vi "SaccadeAnalyser - Main.vi"(8 "error in (no error)":errorcluster, 11 "Data IN":T3={"Impulse Positions"=[{"Start"=5471, "End"=5813, "Impulse Plane"=enum."Yaw", "Impulse Direction +ve?"=FALSE, "Time offset"=0, "Amplitude offset"=0.0}, {"Start"=6974, "End"=7325, "Impulse Plane"=enum."Yaw", "Impulse Direction +ve?"=TRUE, "Time offset"=0, "Amplitude offset"=0.0}, {"Start"=7641, "End"=7980, "Impulse Plane"=enum."Yaw", "Impulse Direction +ve?"=FALSE, "Time offset"=0, "Amplitude offset"=0.0}, {"Start"=9060, "End"=9400, "Impulse Plane"=enum."Yaw", "Impulse Direction +ve?"=FALSE, "Time offset"=0, "Amplitude offset"=0.0}, {"Start"=9938, "End"=10282, "Impulse Plane"=enum."Yaw", "Impulse Direction +ve?"=FALSE, "Time offset"=0, "Amplitude offset"=0.0}, {"Start"=10800, "End"=11142, "Impulse Plane"=enum."Yaw", "Impulse Direction +ve?"=FALSE, "Time offset"=0, "Amplitude offset"=0.0}, {"Start"=11602, "End"=11942, "Impulse Plane"=enum."Yaw", "Impulse Direction +ve?"=TRUE, "Time offset"=0, "Amplitude offset"=0.0}, {"Start"=12449, "End"=12790, "Impulse Plane"=enum."Yaw", "Impulse Direction +ve?"=TRUE, "Time offset"=0, "Amplitude offset"=0.0}, {"Start"=13310, "End"=13653, "Impulse Plane"=enum."Yaw", "Impulse Direction +ve?"=TRUE, "Time offset"=0, "Amplitude offset"=0.0}, {"Start"=14191, "End"=14535, "Impulse Plane"=enum."Yaw", "Impulse Direction +ve?"=TRUE, "Time offset"=0, "Amplitude offset"=0.0}, {"Start"=15040, "End"=15380, "Impulse Plane"=enum."Yaw", "Impulse Direction +ve?"=FALSE, "Time offset"=0, "Amplitude offset"=0.0}, {"Start"=16780, "End"=17124, "Impulse Plane"=enum."Yaw", "Impulse Direction +ve?"=TRUE, "Time offset"=0, "Amplitude offset"=0.0}, {"Start"=17572, "End"=17913, "Impulse Plane"=enum."Yaw", "Impulse Direction +ve?"=FALSE, "Time offset"=0, "Amplitude offset"=0.0}, {"Start"=18369, "End"=18713, "Impulse Plane"=enum."Yaw", "Impulse Direction +ve?"=FALSE, "Time offset"=0, "Amplitude offset"=0.0}, {"Start"=19174, "End"=19519, "Impulse Plane"=enum."Yaw", "Impulse Direction +ve?"=FALSE, "Time offset"=0, "Amplitude offset"=0.0}, {"Start"=19928, "End"=20270, "Impulse Plane"=enum."Yaw", "Impulse Direction +ve?"=TRUE, "Time offset"=0, "Amplitude offset"=0.0}, {"Start"=20762, "End"=21121, "Impulse Plane"=enum."Yaw", "Impulse Direction +ve?"=FALSE, "Time offset"=0, "Amplitude offset"=0.0}, {"Start"=21554, "End"=21888, "Impulse Plane"=enum."Yaw", "Impulse Direction +ve?"=FALSE, "Time offset"=0, "Amplitude offset"=0.0}, {"Start"=22293, "End"=22639, "Impulse Plane"=enum."Yaw", "Impulse Direction +ve?"=TRUE, "Time offset"=0, "Amplitude offset"=0.0}, {"Start"=23109, "End"=23464, "Impulse Plane"=enum."Yaw", "Impulse Direction +ve?"=TRUE, "Time offset"=0, "Amplitude offset"=0.0}, {"Start"=23868, "End"=24215, "Impulse Plane"=enum."Yaw", "Impulse Direction +ve?"=TRUE, "Time offset"=0, "Amplitude offset"=0.0}, {"Start"=24643, "End"=24992, "Impulse Plane"=enum."Yaw", "Impulse Direction +ve?"=FALSE, "Time offset"=0, "Amplitude offset"=0.0}, {"Start"=25685, "End"=26023, "Impulse Plane"=enum."Yaw", "Impulse Direction +ve?"=FALSE, "Time offset"=0, "Amplitude offset"=0.0}, {"Start"=26431, "End"=26768, "Impulse Plane"=enum."Yaw", "Impulse Direction +ve?"=FALSE, "Time offset"=0, "Amplitude offset"=0.0}, {"Start"=27251, "End"=27595, "Impulse Plane"=enum."Yaw", "Impulse Direction +ve?"=FALSE, "Time offset"=0, "Amplitude offset"=0.0}, {"Start"=28832, "End"=29180, "Impulse Plane"=enum."Yaw", "Impulse Direction +ve?"=TRUE, "Time offset"=0, "Amplitude offset"=0.0}, {"Start"=31028, "End"=31383, "Impulse Plane"=enum."LARP", "Impulse Direction +ve?"=FALSE, "Time offset"=0, "Amplitude offset"=0.0}, {"Start"=32603, "End"=32936, "Impulse Plane"=enum."LARP", "Impulse Direction +ve?"=TRUE, "Time offset"=0, "Amplitude offset"=0.0}, {"Start"=33445, "End"=33779, "Impulse Plane"=enum."LARP", "Impulse Direction +ve?"=TRUE, "Time offset"=0, "Amplitude offset"=0.0}, {"Start"=34276, "End"=34629, "Impulse Plane"=enum."LARP", "Impulse Direction +ve?"=FALSE, "Time offset"=0, "Amplitude offset"=0.0}, {"Start"=35114, "End"=35460, "Impulse Plane"=enum."LARP", "Impulse Direction +ve?"=FALSE, "Time offset"=0, "Amplitude offset"=0.0}, {"Start"=35981, "End"=36324, "Impulse Plane"=enum."LARP", "Impulse Direction +ve?"=TRUE, "Time offset"=0, "Amplitude offset"=0.0}, {"Start"=36920, "End"=37249, "Impulse Plane"=enum."LARP", "Impulse Direction +ve?"=TRUE, "Time offset"=0, "Amplitude offset"=0.0}, {"Start"=37988, "End"=38322, "Impulse Plane"=enum."LARP", "Impulse Direction +ve?"=TRUE, "Time offset"=0, "Amplitude offset"=0.0}, {"Start"=38964, "End"=39324, "Impulse Plane"=enum."LARP", "Impulse Direction +ve?"=FALSE, "Time offset"=0, "Amplitude offset"=0.0}, {"Start"=39948, "End"=40284, "Impulse Plane"=enum."LARP", "Impulse Direction +ve?"=TRUE, "Time offset"=0, "Amplitude offset"=0.0}, {"Start"=40958, "End"=41293, "Impulse Plane"=enum."LARP", "Impulse Direction +ve?"=TRUE, "Time offset"=0, "Amplitude offset"=0.0}, {"Start"=41899, "End"=42229, "Impulse Plane"=enum."LARP", "Impulse Direction +ve?"=TRUE, "Time offset"=0, "Amplitude offset"=0.0}, {"Start"=42801, "End"=43154, "Impulse Plane"=enum."LARP", "Impulse Direction +ve?"=FALSE, "Time offset"=0, "Amplitude offset"=0.0}, {"Start"=43641, "End"=43980, "Impulse Plane"=enum."LARP", "Impulse Direction +ve?"=TRUE, "Time offset"=0, "Amplitude offset"=0.0}, {"Start"=44466, "End"=44821, "Impulse Plane"=enum."LARP", "Impulse Direction +ve?"=FALSE, "Time offset"=0, "Amplitude offset"=0.0}, {"Start"=45388, "End"=45722, "Impulse Plane"=enum."LARP", "Impulse Direction +ve?"=TRUE, "Time offset"=0, "Amplitude offset"=0.0}, {"Start"=46149, "End"=46510, "Impulse Plane"=enum."LARP", "Impulse Direction +ve?"=FALSE, "Time offset"=0, "Amplitude offset"=0.0}, {"Start"=47874, "End"=48206, "Impulse Plane"=enum."LARP", "Impulse Direction +ve?"=TRUE, "Time offset"=0, "Amplitude offset"=0.0}, {"Start"=50143, "End"=50479, "Impulse Plane"=enum."RALP", "Impulse Direction +ve?"=TRUE, "Time offset"=0, "Amplitude offset"=0.0}, {"Start"=50976, "End"=51310, "Impulse Plane"=enum."RALP", "Impulse Direction +ve?"=FALSE, "Time offset"=0, "Amplitude offset"=0.0}, {"Start"=51892, "End"=52226, "Impulse Plane"=enum."RALP", "Impulse Direction +ve?"=FALSE, "Time offset"=0, "Amplitude offset"=0.0}, {"Start"=52839, "End"=53171, "Impulse Plane"=enum."RALP", "Impulse Direction +ve?"=FALSE, "Time offset"=0, "Amplitude offset"=0.0}, {"Start"=53676, "End"=54012, "Impulse Plane"=enum."RALP", "Impulse Direction +ve?"=TRUE, "Time offset"=0, "Amplitude offset"=0.0}, {"Start"=54530, "End"=54877, "Impulse Plane"=enum."RALP", "Impulse Direction +ve?"=FALSE, "Time offset"=0, "Amplitude offset"=0.0}, {"Start"=55371, "End"=55711, "Impulse Plane"=enum."RALP", "Impulse Direction +ve?"=TRUE, "Time offset"=0, "Amplitude offset"=0.0}, {"Start"=56153, "End"=56482, "Impulse Plane"=enum."RALP", "Impulse Direction +ve?"=FALSE, "Time offset"=0, "Amplitude offset"=0.0}, {"Start"=57053, "End"=57390, "Impulse Plane"=enum."RALP", "Impulse Direction +ve?"=FALSE, "Time offset"=0, "Amplitude offset"=0.0}, {"Start"=57954, "End"=58292, "Impulse Plane"=enum."RALP", "Impulse Direction +ve?"=FALSE, "Time offset"=0, "Amplitude offset"=0.0}, {"Start"=58794, "End"=59130, "Impulse Plane"=enum."RALP", "Impulse Direction +ve?"=TRUE, "Time offset"=0, "Amplitude offset"=0.0}, {"Start"=59587, "End"=59931, "Impulse Plane"=enum."RALP", "Impulse Direction +ve?"=TRUE, "Time offset"=0, "Amplitude offset"=0.0}, {"Start"=60399, "End"=60744, "Impulse Plane"=enum."RALP", "Impulse Direction +ve?"=FALSE, "Time offset"=0, "Amplitude offset"=0.0}, {"Start"=61218, "End"=61559, "Impulse Plane"=enum."RALP", "Impulse Direction +ve?"=FALSE, "Time offset"=0, "Amplitude offset"=0.0}, {"Start"=62100, "End"=62442, "Impulse Plane"=enum."RALP", "Impulse Direction +ve?"=FALSE, "Time offset"=0, "Amplitude offset"=0.0}, {"Start"=62989, "End"=63322, "Impulse Plane"=enum."RALP", "Impulse Direction +ve?"=FALSE, "Time offset"=0, "Amplitude offset"=0.0}, {"Start"=63787, "End"=64136, "Impulse Plane"=enum."RALP", "Impulse Direction +ve?"=TRUE, "Time offset"=0, "Amplitude offset"=0.0}, {"Start"=64603, "End"=64953, "Impulse Plane"=enum."RALP", "Impulse Direction +ve?"=FALSE, "Time offset"=0, "Amplitude offset"=0.0}, {"Start"=65462, "End"=65795, "Impulse Plane"=enum."RALP", "Impulse Direction +ve?"=FALSE, "Time offset"=0, "Amplitude offset"=0.0}, {"Start"=66308, "End"=66645, "Impulse Plane"=enum."RALP", "Impulse Direction +ve?"=FALSE, "Time offset"=0, "Amplitude offset"=0.0}, {"Start"=67052, "End"=67402, "Impulse Plane"=enum."RALP", "Impulse Direction +ve?"=TRUE, "Time offset"=0, "Amplitude offset"=0.0}], "No. Imp"=15, "Parameter Time Series"=[{"time offset"=0.0, "Offset"=0.0, "Gain"=1.0, "inverse"=FALSE, "filter data"=FALSE, "dots"=FALSE, "interpolate"=FALSE, "List 1"=5, "Color Box"=6618880, "Boolean"=TRUE}, {"time offset"=0.0, "Offset"=0.0, "Gain"=1.0, "inverse"=FALSE, "filter data"=FALSE, "dots"=FALSE, "interpolate"=FALSE, "List 1"=6, "Color Box"=6618880, "Boolean"=FALSE}, {"time offset"=0.0, "Offset"=0.0, "Gain"=1.0, "inverse"=FALSE, "filter data"=FALSE, "dots"=FALSE, "interpolate"=FALSE, "List 1"=7, "Color Box"=6618880, "Boolean"=FALSE}, {"time offset"=0.0, "Offset"=0.0, "Gain"=1.0, "inverse"=FALSE, "filter data"=FALSE, "dots"=FALSE, "interpolate"=FALSE, "List 1"=13, "Color Box"=16777224, "Boolean"=TRUE}, {"time offset"=0.0, "Offset"=0.0, "Gain"=1.0, "inverse"=FALSE, "filter data"=FALSE, "dots"=FALSE, "interpolate"=FALSE, "List 1"=14, "Color Box"=16777224, "Boolean"=FALSE}, {"time offset"=0.0, "Offset"=0.0, "Gain"=1.0, "inverse"=FALSE, "filter data"=FALSE, "dots"=FALSE, "interpolate"=FALSE, "List 1"=15, "Color Box"=16777224, "Boolean"=FALSE}], "Parameter Impuls Series"=[{"Color"=6618880, "Visible"=TRUE, "Channel"=1, "Invert"=FALSE, "Desaccade"=FALSE, "Offset"=0.0, "Gain"=1.0}, {"Color"=6618880, "Visible"=FALSE, "Channel"=6, "Invert"=FALSE, "Desaccade"=FALSE, "Offset"=0.0, "Gain"=1.0}, {"Color"=6618880, "Visible"=FALSE, "Channel"=7, "Invert"=FALSE, "Desaccade"=FALSE, "Offset"=0.0, "Gain"=1.0}, {"Color"=16777224, "Visible"=TRUE, "Channel"=13, "Invert"=FALSE, "Desaccade"=FALSE, "Offset"=0.0, "Gain"=1.0}, {"Color"=16777224, "Visible"=FALSE, "Channel"=14, "Invert"=FALSE, "Desaccade"=FALSE, "Offset"=0.0, "Gain"=1.0}, {"Color"=16777224, "Visible"=FALSE, "Channel"=15, "Invert"=FALSE, "Desaccade"=FALSE, "Offset"=0.0, "Gain"=1.0}], "Experiment Parameters"={"Freq"=0.0, "Vel"=0, "Acc"=0, "Stimulus"="Head Impulse"}, "Autosort File"=refnum, "Data File"={"Data Channels"=array34x71049[2415666 elements], "Sample Rate"=500, "Channel List"=["Hz Position-in-Head", "Hz Velocity-in-Head", "Hy Position-in-Head", "Hy Velocity-in-Head", "Hx Position-in-Head", "Hx Velocity-in-Head", "Hl Velocity-in-Head", "Hr Velocity-in-Head", "Lx Position-in-Head", "Ly Position-in-Head", "Lz Position-in-Head", "Lx Velocity-in-Head", "Ly Velocity-in-Head", "Lz Velocity-in-Head", "Ll Velocity-in-Head", "Lr Velocity-in-Head", "Rx Position-in-Head", "Ry Position-in-Head", "Rz Position-in-Head", "Rx Velocity-in-Head", "Ry Velocity-in-Head", "Rz Velocity-in-Head", "Rl Velocity-in-Head", "Rr Velocity-in-Head", "Target on/off", "aux input 1", "aux input 2", " ", "", "", "", "Target Hor", "Target Ver", ""]}, "Experiment data path"=path "C:/Users/w.figtree/Desktop/Coils Data/3", "Image data path"=path "/Macintosh HD/Users/patrick/Studium/Diploma Thesis/Data Analysis", "LVS data path"=path "/Macintosh HD/Users/patrick/Studium/Diploma Thesis/Data Analysis", "Raw copy path"=path "/Macintosh HD/Users/patrick/Studium/Diploma Thesis/Data Analysis", "filename"="passive_lvs.lvs", "desaccading parameters"={"Tolerance"=3, "Acc Range"=7000.0, "Sample Rate"=500, "Impulse Plane 2"=enum."Yaw", "Impulse dir"=FALSE}, "Experiment Parameters 2"={"Subject"="SE Trial Short Term", "Strain"="", "Rotation plane"="", "Experimenter"=" ", "Trial"=0.0, "Time"=0.0}, "Excel"={"Excel._Application"=refnum, "Use Excel"=TRUE, "Worksheet SINE"=refnum, "Row SINE"=0, "Worksheet TRANS"=refnum, "Row TRANS"=0}, "Session Config File"=refnum, "Autosort Parameter Set"=4, "EMA Version"="EMA 2016a", "desacc "={"Threshold 1 [Acc]"=7000.0, "Threshold 2 [% of TH1]"=60, "tolerance"=3, "Search WD "=0.1, " always use TH2"=FALSE, "Range"=3.0, "Max time"=120.0, "Min time"=20.0, "Velocity Threshold"=150}, "Cycle Nr for Saccades"={"POS"=0, "NEG"=0}, "calibration name"="u_calibration_1_p00001s001_calib.mat", "Excel"=refnum} {"Parameter Time Series"."time offset" format="%.3f"; "Parameter Time Series"."Gain" format="%.1f"; "Parameter Time Series"."Offset" format="%.1f"; "Parameter Time Series"."List 1" items=["Motor-Pos", "Motor-Vel", "Lx Position-in-Head", "Ly Position-in-Head", "Lz Position-in-Head", "Lx Velocity-in-Head", "Ly Velocity-in-Head", "Lz Velocity-in-Head", "Ll Velocity-in-Head", "Lr Velocity-in-Head", "Lx Accel-in-Head", "Ly Accel-in-Head", "Lz Accel-in-Head", "Rx Position-in-Head", "Ry Position-in-Head", "Rz Position-in-Head", "Rx Velocity-in-Head", "Ry Velocity-in-Head", "Rz Velocity-in-Head", "Rl Velocity-in-Head", "Rr Velocity-in-Head", "Rx Accel-in-Head", "Ry Accel-in-Head", "Rz Accel-in-Head", "Global Trigger", "", "", ""]; "Parameter Impuls Series"."Gain" format="%.1f"; "Parameter Impuls Series"."Offset" format="%.1f"}) -> (0 "error out":errorcluster, 3 "Data OUT":T3={"Impulse Positions"=[{"Start"=5471, "End"=5813, "Impulse Plane"=enum."Yaw", "Impulse Direction +ve?"=FALSE, "Time offset"=0, "Amplitude offset"=0.0}, {"Start"=6974, "End"=7325, "Impulse Plane"=enum."Yaw", "Impulse Direction +ve?"=TRUE, "Time offset"=0, "Amplitude offset"=0.0}, {"Start"=7641, "End"=7980, "Impulse Plane"=enum."Yaw", "Impulse Direction +ve?"=FALSE, "Time offset"=0, "Amplitude offset"=0.0}, {"Start"=9060, "End"=9400, "Impulse Plane"=enum."Yaw", "Impulse Direction +ve?"=FALSE, "Time offset"=0, "Amplitude offset"=0.0}, {"Start"=9938, "End"=10282, "Impulse Plane"=enum."Yaw", "Impulse Direction +ve?"=FALSE, "Time offset"=0, "Amplitude offset"=0.0}, {"Start"=10800, "End"=11142, "Impulse Plane"=enum."Yaw", "Impulse Direction +ve?"=FALSE, "Time offset"=0, "Amplitude offset"=0.0}, {"Start"=11602, "End"=11942, "Impulse Plane"=enum."Yaw", "Impulse Direction +ve?"=TRUE, "Time offset"=0, "Amplitude offset"=0.0}, {"Start"=12449, "End"=12790, "Impulse Plane"=enum."Yaw", "Impulse Direction +ve?"=TRUE, "Time offset"=0, "Amplitude offset"=0.0}, {"Start"=13310, "End"=13653, "Impulse Plane"=enum."Yaw", "Impulse Direction +ve?"=TRUE, "Time offset"=0, "Amplitude offset"=0.0}, {"Start"=14191, "End"=14535, "Impulse Plane"=enum."Yaw", "Impulse Direction +ve?"=TRUE, "Time offset"=0, "Amplitude offset"=0.0}, {"Start"=15040, "End"=15380, "Impulse Plane"=enum."Yaw", "Impulse Direction +ve?"=FALSE, "Time offset"=0, "Amplitude offset"=0.0}, {"Start"=16780, "End"=17124, "Impulse Plane"=enum."Yaw", "Impulse Direction +ve?"=TRUE, "Time offset"=0, "Amplitude offset"=0.0}, {"Start"=17572, "End"=17913, "Impulse Plane"=enum."Yaw", "Impulse Direction +ve?"=FALSE, "Time offset"=0, "Amplitude offset"=0.0}, {"Start"=18369, "End"=18713, "Impulse Plane"=enum."Yaw", "Impulse Direction +ve?"=FALSE, "Time offset"=0, "Amplitude offset"=0.0}, {"Start"=19174, "End"=19519, "Impulse Plane"=enum."Yaw", "Impulse Direction +ve?"=FALSE, "Time offset"=0, "Amplitude offset"=0.0}, {"Start"=19928, "End"=20270, "Impulse Plane"=enum."Yaw", "Impulse Direction +ve?"=TRUE, "Time offset"=0, "Amplitude offset"=0.0}, {"Start"=20762, "End"=21121, "Impulse Plane"=enum."Yaw", "Impulse Direction +ve?"=FALSE, "Time offset"=0, "Amplitude offset"=0.0}, {"Start"=21554, "End"=21888, "Impulse Plane"=enum."Yaw", "Impulse Direction +ve?"=FALSE, "Time offset"=0, "Amplitude offset"=0.0}, {"Start"=22293, "End"=22639, "Impulse Plane"=enum."Yaw", "Impulse Direction +ve?"=TRUE, "Time offset"=0, "Amplitude offset"=0.0}, {"Start"=23109, "End"=23464, "Impulse Plane"=enum."Yaw", "Impulse Direction +ve?"=TRUE, "Time offset"=0, "Amplitude offset"=0.0}, {"Start"=23868, "End"=24215, "Impulse Plane"=enum."Yaw", "Impulse Direction +ve?"=TRUE, "Time offset"=0, "Amplitude offset"=0.0}, {"Start"=24643, "End"=24992, "Impulse Plane"=enum."Yaw", "Impulse Direction +ve?"=FALSE, "Time offset"=0, "Amplitude offset"=0.0}, {"Start"=25685, "End"=26023, "Impulse Plane"=enum."Yaw", "Impulse Direction +ve?"=FALSE, "Time offset"=0, "Amplitude offset"=0.0}, {"Start"=26431, "End"=26768, "Impulse Plane"=enum."Yaw", "Impulse Direction +ve?"=FALSE, "Time offset"=0, "Amplitude offset"=0.0}, {"Start"=27251, "End"=27595, "Impulse Plane"=enum."Yaw", "Impulse Direction +ve?"=FALSE, "Time offset"=0, "Amplitude offset"=0.0}, {"Start"=28832, "End"=29180, "Impulse Plane"=enum."Yaw", "Impulse Direction +ve?"=TRUE, "Time offset"=0, "Amplitude offset"=0.0}, {"Start"=31028, "End"=31383, "Impulse Plane"=enum."LARP", "Impulse Direction +ve?"=FALSE, "Time offset"=0, "Amplitude offset"=0.0}, {"Start"=32603, "End"=32936, "Impulse Plane"=enum."LARP", "Impulse Direction +ve?"=TRUE, "Time offset"=0, "Amplitude offset"=0.0}, {"Start"=33445, "End"=33779, "Impulse Plane"=enum."LARP", "Impulse Direction +ve?"=TRUE, "Time offset"=0, "Amplitude offset"=0.0}, {"Start"=34276, "End"=34629, "Impulse Plane"=enum."LARP", "Impulse Direction +ve?"=FALSE, "Time offset"=0, "Amplitude offset"=0.0}, {"Start"=35114, "End"=35460, "Impulse Plane"=enum."LARP", "Impulse Direction +ve?"=FALSE, "Time offset"=0, "Amplitude offset"=0.0}, {"Start"=35981, "End"=36324, "Impulse Plane"=enum."LARP", "Impulse Direction +ve?"=TRUE, "Time offset"=0, "Amplitude offset"=0.0}, {"Start"=36920, "End"=37249, "Impulse Plane"=enum."LARP", "Impulse Direction +ve?"=TRUE, "Time offset"=0, "Amplitude offset"=0.0}, {"Start"=37988, "End"=38322, "Impulse Plane"=enum."LARP", "Impulse Direction +ve?"=TRUE, "Time offset"=0, "Amplitude offset"=0.0}, {"Start"=38964, "End"=39324, "Impulse Plane"=enum."LARP", "Impulse Direction +ve?"=FALSE, "Time offset"=0, "Amplitude offset"=0.0}, {"Start"=39948, "End"=40284, "Impulse Plane"=enum."LARP", "Impulse Direction +ve?"=TRUE, "Time offset"=0, "Amplitude offset"=0.0}, {"Start"=40958, "End"=41293, "Impulse Plane"=enum."LARP", "Impulse Direction +ve?"=TRUE, "Time offset"=0, "Amplitude offset"=0.0}, {"Start"=41899, "End"=42229, "Impulse Plane"=enum."LARP", "Impulse Direction +ve?"=TRUE, "Time offset"=0, "Amplitude offset"=0.0}, {"Start"=42801, "End"=43154, "Impulse Plane"=enum."LARP", "Impulse Direction +ve?"=FALSE, "Time offset"=0, "Amplitude offset"=0.0}, {"Start"=43641, "End"=43980, "Impulse Plane"=enum."LARP", "Impulse Direction +ve?"=TRUE, "Time offset"=0, "Amplitude offset"=0.0}, {"Start"=44466, "End"=44821, "Impulse Plane"=enum."LARP", "Impulse Direction +ve?"=FALSE, "Time offset"=0, "Amplitude offset"=0.0}, {"Start"=45388, "End"=45722, "Impulse Plane"=enum."LARP", "Impulse Direction +ve?"=TRUE, "Time offset"=0, "Amplitude offset"=0.0}, {"Start"=46149, "End"=46510, "Impulse Plane"=enum."LARP", "Impulse Direction +ve?"=FALSE, "Time offset"=0, "Amplitude offset"=0.0}, {"Start"=47874, "End"=48206, "Impulse Plane"=enum."LARP", "Impulse Direction +ve?"=TRUE, "Time offset"=0, "Amplitude offset"=0.0}, {"Start"=50143, "End"=50479, "Impulse Plane"=enum."RALP", "Impulse Direction +ve?"=TRUE, "Time offset"=0, "Amplitude offset"=0.0}, {"Start"=50976, "End"=51310, "Impulse Plane"=enum."RALP", "Impulse Direction +ve?"=FALSE, "Time offset"=0, "Amplitude offset"=0.0}, {"Start"=51892, "End"=52226, "Impulse Plane"=enum."RALP", "Impulse Direction +ve?"=FALSE, "Time offset"=0, "Amplitude offset"=0.0}, {"Start"=52839, "End"=53171, "Impulse Plane"=enum."RALP", "Impulse Direction +ve?"=FALSE, "Time offset"=0, "Amplitude offset"=0.0}, {"Start"=53676, "End"=54012, "Impulse Plane"=enum."RALP", "Impulse Direction +ve?"=TRUE, "Time offset"=0, "Amplitude offset"=0.0}, {"Start"=54530, "End"=54877, "Impulse Plane"=enum."RALP", "Impulse Direction +ve?"=FALSE, "Time offset"=0, "Amplitude offset"=0.0}, {"Start"=55371, "End"=55711, "Impulse Plane"=enum."RALP", "Impulse Direction +ve?"=TRUE, "Time offset"=0, "Amplitude offset"=0.0}, {"Start" (continued)
-54.18247144797069, -58.85281689160722, -63.91527138905126, -69.3816768064082, -75.22429125556431, -81.37762698666069, -87.75180274500077, -94.23796057331468, -100.71571205715665, -107.07112629665112, -113.2080026001733, -119.04423669102385, -124.52204306435647, -129.6179037571645, -134.3434864691834, -138.73926124919257, -142.86209314608806, -146.77852632236662, -150.55410864602925, -154.2421058778206, -157.8608435457303, -161.38556543542902, -164.75519586867193, -167.878112041269, -170.6502845196639, -172.96947690993014, -174.74780026444301, -175.9280234619177, -176.49581974428241, -176.47783870432215, -175.92566673674776, -174.9055756754708, -173.49760575715453, -171.7834624665382, -169.83161630071703, -167.69551193456192, -165.41647407002708, -163.02092536825774, -160.50399517975018, -157.8263795045505, -154.92869248428667, -151.7392178656919, -148.18363503277277, -144.19520813467358, -139.7423154139475, -134.85092284147765, -129.5970332835845, -124.096932573479, -118.48663287415354, -112.89326377420801, -107.41192289509742, -102.09133956405964, -96.91932930045344, -91.82924084415812, -86.72929490339284, -81.52158361787951, -76.1282941909947, -70.50762789188907, -64.66023923119536, -58.64052733673002, -52.54018902245833, -46.45809012434801, -40.486829092171924, -34.70668063780862, -29.173216331551032, -23.9068786063661, -18.897099148136192, -14.114118816191809, -9.520293557801804, -5.085847473387664, -0.7981606818145077, 3.3266043290818934, 7.243600002532165, 10.885420249895338, 14.161767360680157, 16.984238540492136, 19.291750959591102, 21.063902044408295, 22.331979940494904, 23.17761342325074, 23.721961474588795, 24.112784288313726, 24.491300668844953, 24.954722286655777, 25.548108319995535, 26.25835502219787, 27.009352039914436, 27.685557314658922, 28.168888441777447, 28.373084425112715, 28.259535186152696, 27.842133775360793, 27.188150755230232, 26.406250500356492, 25.615461263548987, 24.910485897492496, 24.346023233855814, 23.92691315712331, 23.608231595379664, 23.316584778717154, 22.97439243815799, 22.516811117961932, 21.918073580662337, 21.199324383617018, 20.41268969980475, 19.630359806325515, 18.925688883278173, 18.35445806189755, 17.94200024522094, 17.668844949225154, 17.48230912370444, 17.320743177459768, 17.12385592094169, 16.848651342354945, 16.48521549632595, 16.053715760638944, 15.599731481783138, 15.187115328471895, 14.872560249314708, 14.690476111081628, 14.654617574216875, 14.750456991166905, 14.93679615927241, 15.155141464873388, 15.333160190841902, 15.398738035467435, 15.29496106484143, 14.988709233052518, 14.477914274794113, 13.791715142798871, 12.98608736614728, 12.143907008543643, 11.359534797804809, 10.712039410503696, 10.254402747409266, 9.996473345954591, 9.896879988642478, 9.883403069720273, 9.859589516965436, 9.721973952789982, 9.396474330493742, 8.8572878573063, 8.126364534227164, 7.264175814803053, 6.355998470318044, 5.489439194352843, 4.7331879614108505, 4.122707511796716, 3.65264371887878, 3.286290193278276, 2.9766469769695836, 2.680197842403923, 2.3715537962781688, 2.054470430273149, 1.7588126482498483, 1.52762158204097, 1.3969988798953015, 1.3837046107842852, 1.4780084889263279, 1.6331366871599418, 1.7862480312450515, 1.885768730098075, 1.8964541688469012, 1.8162169165165416, 1.6814817264069895, 1.5492834774423194, 1.484862531012908, 1.5421064788750378, 1.7350747823148893, 2.0342448608033195, 2.379446691066832, 2.6948282712623737, 2.911116060608993, 2.9842378047308706, 2.9083083080686016, 2.7160208417143217, 2.4711098156462157, 2.256715447981385, 2.148013016215092, 2.187585248222959, 2.3803037826910867, 2.6983328403827826, 3.0862430081882692, 3.4771760047328684, 3.8144998017781937, 4.063608708587875, 4.220732678012546, 4.314758958249271, 4.385161364394381, 4.451563149829603, 4.516553485433068, 4.5711222556517725, 4.5789244340039374, 4.495990520342794, 4.300879185323019, 3.999300290032796, 3.6267710749586684, 3.2456696612949933, 2.9267834631551075, 2.7279329460099753, 2.6791526464304543, 2.764403437378572, 2.924982772356076, 3.0845635011921093, 3.1660247683184704, 3.1140733546638995, 2.9142235252131066, 2.6045926121551446, 2.264439578758724, 1.9827108041327461, 1.8446572231616623, 1.9016973069974075, 2.1477989186114366, 2.527543767369518, 2.9494945166396676, 3.316294504066529, 3.554920234020117, 3.6294412691334976, 3.5518308896879076, 3.381651807861633, 3.1987672126172613, 3.0794265856609844, 3.076618052634122, 3.2028855967548573, 3.4357915499468694, 3.7262128069143348, 4.011008721689602, 4.241013746798439, 4.4004494908201375, 4.501263210760912, 4.57564361728543, 4.674574896548988, 4.847554015003683, 5.118620024272339, 5.476792247776838, 5.882038540567098, 6.280337746221127, 6.610772610856507, 6.824568969574903, 6.902440280843165, 6.859370359784798, 6.743336212454451, 6.611463939269871, 6.5152928701361645]}, {[0.0, 2.0, 4.0, 6.0, 8.0, 10.0, 12.0, 14.0, 16.0, 18.000000000000004, 20.0, 22.0, 24.0, 26.000000000000004, 28.0, 30.0, 32.0, 34.0, 36.00000000000001, 38.0, 40.0, 42.0, 44.0, 46.0, 48.0, 50.0, 52.00000000000001, 54.0, 56.0, 58.0, 60.0, 62.0, 64.0, 66.0, 68.0, 70.0, 72.00000000000001, 74.0, 76.0, 78.0, 80.0, 82.0, 84.0, 86.0, 88.0, 90.0, 92.0, 94.0, 96.0, 98.0, 100.0, 102.00000000000001, 104.00000000000001, 106.0, 108.0, 110.0, 112.0, 114.0, 116.0, 118.00000000000001, 120.0, 122.0, 124.0, 126.0, 128.0, 130.0, 132.0, 134.0, 136.0, 138.0, 140.0, 142.00000000000003, 144.00000000000003, 146.0, 148.0, 150.0, 152.0, 154.0, 156.0, 158.0, 160.0, 162.0, 164.0, 166.0, 168.0, 170.0, 172.0, 174.00000000000003, 176.0, 178.0, 180.0, 182.0, 184.0, 186.0, 188.0, 190.0, 192.0, 194.0, 196.0, 198.0, 200.0, 202.0, 204.00000000000003, 206.00000000000003, 208.00000000000003, 210.0, 212.0, 214.0, 216.0, 218.0, 220.0, 222.0, 224.0, 226.0, 228.0, 230.0, 232.0, 234.0, 236.00000000000003, 238.00000000000003, 240.0, 242.0, 244.0, 246.0, 248.0, 250.0, 252.0, 254.0, 256.0, 258.0, 260.0, 262.0, 264.0, 266.0, 268.0, 270.0, 272.0, 274.0, 276.0, 278.0, 280.0, 282.0, 284.00000000000006, 286.00000000000006, 288.00000000000006, 290.0, 292.0, 294.0, 296.0, 298.0, 300.0, 302.0, 304.0, 306.0, 308.0, 310.0, 312.0, 314.0, 316.0, 318.0, 320.0, 322.0, 324.0, 326.0, 328.0, 330.0, 332.0, 334.0, 336.0, 338.0, 340.0, 342.0, 344.0, 346.00000000000006, 348.00000000000006, 350.00000000000006, 352.0, 354.0, 356.0, 358.0, 360.0, 362.0, 364.0, 366.0, 368.0, 370.0, 372.0, 374.0, 376.0, 378.0, 380.0, 382.0, 384.0, 386.0, 388.0, 390.0, 392.0, 394.0, 396.0, 398.0, 400.0, 402.0, 404.0, 406.0, 408.00000000000006, 410.00000000000006, 412.00000000000006, 414.00000000000006, 416.00000000000006, 418.0, 420.0, 422.0, 424.0, 426.0, 428.0, 430.0, 432.0, 434.0, 436.0, 438.0, 440.0, 442.0, 444.0, 446.0, 448.0, 450.0, 452.0, 454.0, 456.0, 458.0, 460.0, 462.0, 464.0, 466.0, 468.0, 470.00000000000006, 472.00000000000006, 474.00000000000006, 476.00000000000006, 478.00000000000006, 480.0, 482.0, 484.0, 486.0, 488.0, 490.0, 492.0, 494.0, 496.0, 498.0, 500.0, 502.0, 504.0, 506.0, 508.0, 510.0, 512.0, 514.0, 516.0, 518.0, 520.0, 522.0, 524.0, 526.0, 528.0, 530.0, 532.0, 534.0, 536.0, 538.0, 540.0, 542.0, 544.0, 546.0, 548.0, 550.0, 552.0, 554.0, 556.0, 558.0, 560.0, 562.0, 564.0, 566.0000000000001, 568.0000000000001, 570.0000000000001, 572.0000000000001, 574.0000000000001, 576.0000000000001, 578.0, 580.0, 582.0, 584.0, 586.0, 588.0, 590.0, 592.0, 594.0, 596.0, 598.0, 600.0, 602.0, 604.0, 606.0, 608.0, 610.0, 612.0, 614.0, 616.0, 618.0, 620.0, 622.0, 624.0, 626.0, 628.0, 630.0, 632.0, 634.0, 636.0, 638.0, 640.0, 642.0, 644.0, 646.0, 648.0, 650.0, 652.0, 654.0, 656.0, 658.0, 660.0, 662.0, 664.0, 666.0, 668.0], [0.5652055469945032, 0.4509292345615292, 0.29146525563787096, 0.11608355051525354, -0.03944427627728064, -0.14425899395826725, -0.18641372541902768, -0.17724549418876112, -0.14875549408117994, -0.13979642339051845, -0.17639297227747086, -0.2618215747145207, -0.37736442963764105, -0.48966535649601717, -0.564165046890392, -0.5737251668598837, -0.5101821643194544, -0.40476573043766173, -0.3213937689303359, -0.32918741736212453, -0.47542626078155603, -0.7718148834308742, -1.1836147403547979, -1.6232197179595114, -1.978819866124418, -2.141492054575065, -2.0328624108660147, -1.642501637330545, -1.0338876507156414, -0.3270373925701824, 0.3279989632620812, 0.7950752074096783, 0.9957684246360421, 0.9286281158278258, 0.6685838673402991, 0.34670241014339753, 0.10573889712230322, 0.05547558404689745, 0.23976459287755425, 0.6140761216406156, 1.055025860048497, 1.4001841012543323, 1.4953665633641169, 1.2454781539501738, 0.6579242213265637, -0.16801224570884443, -1.066354412369801, -1.8217804712171102, -2.240836065536339, -2.205391656968313, -1.6869713932536996, -0.7533243250730095, 0.4495431074931133, 1.7280511717826315, 2.894410022913668, 3.807643774945902, 4.387602574804731, 4.628908676296568, 4.587612085165617, 4.351271533197959, 4.019980861910334, 3.6875018760990983, 3.424065239817402, 3.265247155816361, 3.2149478764447252, 3.267136690424657, 3.424531246903072, 3.6865000308570295, 4.050993530196079, 4.5290844264875485, 5.130962664057412, 5.85631427504533, 6.691971633646059, 7.616074568235852, 8.600493973058672, 9.618010673917222, 10.654735601996428, 11.706730511694701, 12.785661199875143, 13.921911797611834, 15.151776289586373, 16.512269106070725, 18.03525488942543, 19.74007555337839, 21.638277130741677, 23.729914870124073, 26.001287762510927, 28.448519824529463, 31.090537701618505, 33.96460423688153, 37.13237306835261, 40.677411856769766, 44.68007078378511, 49.19985342949783, 54.273312223776145, 59.88527276239272, 65.95824383010901, 72.37866570458567, 79.00418724344567, 85.68890263088662, 92.30470439865232, 98.75229088834524, 104.97957991508198, 110.97546699511481, 116.77272780388314, 122.43750400493667, 128.04419410667253, 133.67154937587003, 139.3878720556421, 145.23089245467895, 151.20395470208942, 157.271344466521, 163.35789560721776, 169.35486103682769, 175.11471555911692, 180.47081695075735, 185.27417608584693, 189.40335057538567, 192.774986737542, 195.3605336700389, 197.19606785789853, 198.3655099634007, 198.96666339078575, 199.09922192598594, 198.84211620809415, 198.2228362952137, 197.2073592222402, 195.7095577445869, 193.61931618204414, 190.82566973049552, 187.23422375307103, 182.78727889114754, 177.47504314355393, 171.33279951087175, 164.43472688551492, 156.87857461810503, 148.76847213682646, 140.22359594749082, 131.37074386903743, 122.33322260721471, 113.24079454210826, 104.22373615250909, 95.39229256586161, 86.82050771485542, 78.54621815654232, 70.56062254642123, 62.80184837235152, 55.18771607765946, 47.643548359447266, 40.12386670389399, 32.63244543069931, 25.22409164511008, 17.997611977681387, 11.070577244465808, 4.562222599262982, -1.4334655711773734, -6.873162958747107, -11.757498725288368, -16.121589615802073, -20.02486933976549, -23.5277086834347, -26.669700293136763, -29.467784171689594, -31.914867063085026, -33.998146720198235, -35.711154782934976, -37.05066071012995, -38.03591636026024, -38.709837605979786, -39.12512759743504, -39.32697872162574, -39.33945090439231, -39.166137933870985, -38.788065765308964, -38.168940088655, -37.26909821875877, -36.06742645162676, -34.57372866514956, -32.822579990667805, -30.870646914619496, -28.798348698799614, -26.69711452920234, -24.639877983567146, -22.68419564375953, -20.878936376239324, -19.24419272671362, -17.77397109947476, -16.434404928584506, -15.169389984551167, -13.91752976368609, -12.615863301860433, -11.208415401935262, -9.66295225071839, -7.9929528202837705, -6.24570779382055, -4.48837373627782, -2.8126036934657, -1.309299667373761, -0.04842051847741757, 0.9280938622794856, 1.6150405400117656, 2.0336981296897143, 2.2163781550294672, 2.2025217689841057, 2.042027537222708, 1.778209771811973, 1.4361198783417137, 1.0410833515742723, 0.6302257668770679, 0.2348275616761697, -0.13027684860060162, -0.45052503219589823, -0.719968311724827, -0.9477830313772344, -1.1610584493581797, -1.41167471274413, -1.7517181843749619, -2.2216191689314897, -2.8505282324621106, -3.647049339970998, -4.595458808716646, -5.654265790554243, -6.7600403449839686, -7.845827174911193, -8.850022144362535, -9.717466555813978, -10.411984064929317, -10.917018869743522, -11.230153578680078, -11.362367960195675, -11.337503451820709, -11.191461917349352, -10.959073347599952, -10.676802773919643, -10.39000165158323, -10.136446748900555, -9.94436877133468, -9.832354427664432, -9.804225976871743, -9.848361056025265, -9.935496441759469, -10.018662398352467, -10.037202680162046, -9.93852200612768, -9.684740274177624, -9.254159042418237, -8.659971551770251, -7.951649831532783, -7.2041103868258585, -6.498772617674496, -5.904175129207042, -5.468180989586604, -5.209286754003118, -5.106106814625076, -5.099760199142267, -5.118759729967089, -5.100436464213749, -4.994877785059846, -4.765735595006401, -4.405324822645047, -3.944317446417565, -3.430145900188043, -2.9147319671720338, -2.4456707465567615, -2.0603379466555496, -1.7924346967634288, -1.6580146736480146, -1.6440640700311289, -1.7154623466941208, -1.8281017492398877, -1.9384376159235448, -2.0052622425037447, -1.9970686281196495, -1.9087109827403512, -1.7623526337565631, -1.59843440834224, -1.469698664032985, -1.4231845371415006, -1.4807277350667225, -1.629009460768653, -1.8188062632528441, -1.9742323796249868, -2.0240079408016673, -1.9321348393154623, -1.71157182802277, -1.4360024379154281, -1.2272664562648163, -1.2220473390800324, -1.5291287202479276, -2.185897315036751, -3.1391990564353716, -4.2457757136204215, -5.296213441966732, -6.066579766615599, -6.381392825612332, -6.166036645449278, -5.46483177075599, -4.434995427476712, -3.3174201425682517, -2.371942086222576, -1.8133430513278492, -1.7678218395091205, -2.2435836999764804, -3.127991766060479, -4.223075001633013, -5.302919935465798, -6.1631374951731805, -6.665317720130105, -6.761970656573431, -6.500509128184466, -6.014118865213065, -5.476249324503655, -5.043482754462778, -4.824296641030755, -4.865394734240293, -5.140174934652006, -5.554567410338771, -5.979046786201711, -6.2828067112979795, -6.363957422246631, -6.175029334873952, -5.725364395716184, -5.086683076243041, -4.389436944029693, -3.784042417310893, -3.4068370617572654, -3.3631565997774118, -3.706216715085265, -4.416197133559475, -5.405361378742459, -6.528603008890733, -7.606448710681499, -8.47873739267919, -9.033980228340303]}, {[0.0, 2.0, 4.0, 6.0, 8.0, 10.0, 12.0, 14.0, 16.0, 18.000000000000004, 20.0, 22.0, 24.0, 26.000000000000004, 28.0, 30.0, 32.0, 34.0, 36.00000000000001, 38.0, 40.0, 42.0, 44.0, 46.0, 48.0, 50.0, 52.00000000000001, 54.0, 56.0, 58.0, 60.0, 62.0, 64.0, 66.0, 68.0, 70.0, 72.00000000000001, 74.0, 76.0, 78.0, 80.0, 82.0, 84.0, 86.0, 88.0, 90.0, 92.0, 94.0, 96.0, 98.0, 100.0, 102.00000000000001, 104.00000000000001, 106.0, 108.0, 110.0, 112.0, 114.0, 116.0, 118.00000000000001, 120.0, 122.0, 124.0, 126.0, 128.0, 130.0, 132.0, 134.0, 136.0, 138.0, 140.0, 142.00000000000003, 144.00000000000003, 146.0, 148.0, 150.0, 152.0, 154.0, 156.0, 158.0, 160.0, 162.0, 164.0, 166.0, 168.0, 170.0, 172.0, 174.00000000000003, 176.0, 178.0, 180.0, 182.0, 184.0, 186.0, 188.0, 190.0, 192.0, 194.0, 196.0, 198.0, 200.0, 202.0, 204.00000000000003, 206.00000000000003, 208.00000000000003, 210.0, 212.0, 214.0, 216.0, 218.0, 220.0, 222.0, 224.0, 226.0, 228.0, 230.0, 232.0, 234.0, 236.00000000000003, 238.00000000000003, 240.0, 242.0, 244.0, 246.0, 248.0, 250.0, 252.0, 254.0, 256.0, 258.0, 260.0, 262.0, 264.0, 266.0, 268.0, 270.0, 272.0, 274.0, 276.0, 278.0, 280.0, 282.0, 284.00000000000006, 286.00000000000006, 288.00000000000006, 290.0, 292.0, 294.0, 296.0, 298.0, 300.0, 302.0, 304.0, 306.0, 308.0, 310.0, 312.0, 314.0, 316.0, 318.0, 320.0, 322.0, 324.0, 326.0, 328.0, 330.0, 332.0, 334.0, 336.0, 338.0, 340.0, 342.0, 344.0, 346.00000000000006, 348.00000000000006, 350.00000000000006, 352.0, 354.0, 356.0, 358.0, 360.0, 362.0, 364.0, 366.0, 368.0, 370.0, 372.0, 374.0, 376.0, 378.0, 380.0, 382.0, 384.0, 386.0, 388.0, 390.0, 392.0, 394.0, 396.0, 398.0, 400.0, 402.0, 404.0, 406.0, 408.00000000000006, 410.00000000000006, 412.00000000000006, 414.00000000000006, 416.00000000000006, 418.0, 420.0, 422.0, 424.0, 426.0, 428.0, 430.0, 432.0, 434.0, 436.0, 438.0, 440.0, 442.0, 444.0, 446.0, 448.0, 450.0, 452.0, 454.0, 456.0, 458.0, 460.0, 462.0, 464.0, 466.0, 468.0, 470.00000000000006, 472.00000000000006, 474.00000000000006, 476.00000000000006, 478.00000000000006, 480.0, 482.0, 484.0, 486.0, 488.0, 490.0, 492.0, 494.0, 496.0, 498.0, 500.0, 502.0, 504.0, 506.0, 508.0, 510.0, 512.0, 514.0, 516.0, 518.0, 520.0, 522.0, 524.0, 526.0, 528.0, 530.0, 532.0, 534.0, 536.0, 538.0, 540.0, 542.0, 544.0, 546.0, 548.0, 550.0, 552.0, 554.0, 556.0, 558.0, 560.0, 562.0, 564.0, 566.0000000000001, 568.0000000000001, 570.0000000000001, 572.0000000000001, 574.0000000000001, 576.0000000000001, 578.0, 580.0, 582.0, 584.0, 586.0, 588.0, 590.0, 592.0, 594.0, 596.0, 598.0, 600.0, 602.0, 604.0, 606.0, 608.0, 610.0, 612.0, 614.0, 616.0, 618.0, 620.0, 622.0, 624.0, 626.0, 628.0, 630.0, 632.0, 634.0, 636.0, 638.0, 640.0, 642.0, 644.0, 646.0, 648.0, 650.0, 652.0, 654.0, 656.0, 658.0, 660.0, 662.0, 664.0, 666.0, 668.0], [0.03948487033054526, 0.0395825900730058, 0.02713644331793974, 0.004161878880751146, -0.027768004024055326, -0.06706511491539002, -0.10699191698467247, -0.13483903201683267, -0.1316707374415529, -0.08017936460608288, 0.023143927013765442, 0.16445817376007899, 0.31641155304333246, 0.4456293575171597, 0.5210671650146823, 0.520938020727133, 0.44558688208101893, 0.3346092943170502, 0.2536351645518917, 0.2670362446200141, 0.4231748720735804, 0.7345335004286722, 1.1623298689164079, 1.6194327950015237, 1.9897889478366138, 2.159835176077059, 2.0529025553441094, 1.6558633083515568, 1.0288336751670744, 0.2936481421584247, -0.39380627929476275, -0.8874460091538916, -1.0970604359021796, -1.0105496086899175, -0.6969416896946065, -0.29066040456426867, 0.05062685919433596, 0.19091181886319486, 0.05225275015494102, -0.35574724064872676, -0.9373047839746018, -1.5421224046372908, -2.0067859262610153, -2.2036966364076562, -2.0851674418529953, -1.6864463441418014, -1.1127808809258681, -0.5296567511755885, -0.10474541472351895, 0.04218547373058712, -0.14884321776969855, -0.6637364276012327, -1.4165322653384749, -2.269964974342404, -3.07842649995985, -3.7226939071848832, -4.123710967442161, -4.261982220755737, -4.172333068046154, -3.9233278868141888, -3.6053853104788445, -3.314492021546016, -3.1332262073191615, -3.1135136806254025, -3.2719112367324996, -3.6039116605077055, -4.098358109042088, -4.725208893343449, -5.441126625731933, -6.211450866324668, -7.005150113960987, -7.7929473795155175, -8.547256092914154, -9.250675324005456, -9.904029053084706, -10.519714157671736, -11.122669426527388, -11.751200651980156, -12.454844050419489, -13.288476710419836, -14.299780251921902, -15.522864195183864, -16.979522114418437, -18.67753274196494, -20.60960559186061, -22.75548356194932, -25.08645969146879, -27.586215719552357, -30.2658658742428, -33.15824949599187, -36.32207155039271, -39.841355336077314, -43.80104793755666, -48.272173340568244, -53.30385892736406, -58.89607173541701, -64.99210330722595, -71.49465745995099, -78.27066185779526, -85.17227973788198, -92.05933797250894, -98.81048381117657, -105.33877817935411, -111.59590141588706, -117.57914670998028, -123.32211676945946, -128.8745009426899, -134.29507955385418, -139.63432986948746, -144.9144566767209, -150.11864627827356, -155.18591984565973, -160.01594057192526, -164.48352011417342, -168.4465418336565, -171.76390472050772, -174.33304027143691, -176.1026526206232, -177.07281319835766, -177.30175607852462, -176.90098763503002, -176.01006635319737, -174.76388248431937, -173.27653055693756, -171.6190068657425, -169.8010064991298, -167.77355353506405, -165.44149958342896, -162.69221448272677, -159.4218552710808, -155.55079473775606, -151.03395821320828, -145.8685168405854, -140.08729467736453, -133.7402796055532, -126.87974500591224, -119.54901066636218, -111.7904781325743, -103.64968722277284, 